vi "Dresden R2R Sputter 03.02.2018 IY24.vi"() -> ()   [LabVIEW 2009] (continued)
                                tunnel: [FALSE TRUE] -> w23599
                                frame #0 {
                                n20852 = local write "Ch3_Ch_vbv_do"(TRUE ("Ch1_Ch_cc_on_off_di")) -> ()
                                n20853 = Wait Until Next ms Multiple(millisecond multiple=u32 500) -> ()  [unwired: 1 out]
                                }
                                frame #1 {
                                }
                                }
                                n20854 = local read "Semi"() -> (w23600:bool)
                                n20855 = Or(x=w23599, y=w23600) -> (x .or. y?=w23598:bool)
                                }
                                }
                                frame #1 {
                                }
                                }
                                }
                                frame #1 {
                                n20856 = local read "Semi"() -> (w23610:bool)
                                n20857 = case shown="False" w23610 {
                                frame #0 {
                                n20858 = local write "Ch3_Sd13"(TRUE ("Ch1_Sd12")) -> ()
                                n20859 = Wait (ms)(milliseconds to wait=u32 1000) -> ()  [unwired: 1 out]
                                }
                                frame #1 {
                                }
                                }
                                }
                                }
                                }
                                frame #1 {
                                }
                                }
                                }
                                }
                              }
                              frame #13 {
                                # "TRNS GV-BP2 OPEN"
                                n20860 = local read "Yes 3"() -> (w23613:bool)
                                n20861 = case shown="True" w23613 {
                                frame #0 {
                                }
                                frame #1 {
                                n20862 = local read "Semi"() -> (w23614:bool)
                                n20863 = case shown="False" w23614 {
                                frame #0 {
                                n20864 = stacked-sequence {
                                frame #0 {
                                n20865 = local read "Semi"() -> (w23615:bool)
                                n20866 = case shown="False" w23615 {
                                frame #0 {
                                n20867 = while {
                                i -> [w23623]
                                stop <- w23620 stop-if-true
                                n20868 = Greater?(x=w23623, y=800) -> (0:w23622:bool)
                                n20869 = case shown="True" w23622 {
                                frame #0 {
                                }
                                frame #1 {
                                n20870 = local write "Error Message"("Shut Down process was cancelled.\nPlease check Trns GV-BP2\n connections." ("Error Message")) -> ()
                                n20871 = local write "Semi"(TRUE ("Semi")) -> ()
                                }
                                }
                                n20872 = local read "Ch3_pressure"() -> (w23618:dbl)
                                n20873 = Greater Or Equal?(x=w23618, y=700.0) -> (x >= y?=w23616:bool)
                                n20874 = case shown="True" w23616 {
                                tunnel: [FALSE w23627] -> w23619
                                frame #0 {
                                n20875 = Wait Until Next ms Multiple(millisecond multiple=u32 500) -> ()  [unwired: 1 out]
                                }
                                frame #1 {
                                n20876 = local read "Ch3_Trns_gv_bp2_di"() -> (w23628:bool)
                                n20877 = case shown="False" w23628 {
                                tunnel: [FALSE TRUE] -> w23627
                                frame #0 {
                                n20878 = local write "Ch3_Trns_gv_bp2_do"(TRUE ("Ch1_Trns_gv_bp2_do")) -> ()
                                n20879 = Wait Until Next ms Multiple(millisecond multiple=u32 500) -> ()  [unwired: 1 out]
                                }
                                frame #1 {
                                }
                                }
                                }
                                }
                                n20880 = local read "Semi"() -> (w23621:bool)
                                n20881 = Or(x=w23619, y=w23621) -> (x .or. y?=w23620:bool)
                                }
                                }
                                frame #1 {
                                }
                                }
                                }
                                frame #1 {
                                n20882 = local read "Semi"() -> (w23635:bool)
                                n20883 = case shown="False" w23635 {
                                frame #0 {
                                n20884 = local write "Ch3_Sd14"(TRUE ("Ch2_Sd0 14")) -> ()
                                n20885 = Wait (ms)(milliseconds to wait=u32 1000) -> ()  [unwired: 1 out]
                                }
                                frame #1 {
                                }
                                }
                                }
                                frame #2 {
                                n20886 = local read "Semi"() -> (w23638:bool)
                                n20887 = case shown="False" w23638 {
                                frame #0 {
                                n20888 = Wait (ms)(milliseconds to wait=u32 2000) -> ()  [unwired: 1 out]
                                }
                                frame #1 {
                                }
                                }
                                }
                                }
                                }
                                frame #1 {
                                }
                                }
                                }
                                }
                              }
                              frame #14 {
                                # "TRNS GV-BP OPEN"
                                n20889 = local read "Yes 3"() -> (w23640:bool)
                                n20890 = case shown="True" w23640 {
                                frame #0 {
                                }
                                frame #1 {
                                n20891 = local read "Semi"() -> (w23641:bool)
                                n20892 = case shown="False" w23641 {
                                frame #0 {
                                n20893 = stacked-sequence {
                                frame #0 {
                                n20894 = local read "Semi"() -> (w23642:bool)
                                n20895 = case shown="False" w23642 {
                                frame #0 {
                                n20896 = while {
                                i -> [w23650]
                                stop <- w23647 stop-if-true
                                n20897 = Greater?(x=w23650, y=800) -> (0:w23649:bool)
                                n20898 = case shown="True" w23649 {
                                frame #0 {
                                }
                                frame #1 {
                                n20899 = local write "Error Message"("Shut Down process was cancelled.\nPlease check Trns GV-BP\n connections." ("Error Message")) -> ()
                                n20900 = local write "Semi"(TRUE ("Semi")) -> ()
                                }
                                }
                                n20901 = local read "Ch3_pressure"() -> (w23645:dbl)
                                n20902 = Greater Or Equal?(x=w23645, y=700.0) -> (x >= y?=w23643:bool)
                                n20903 = case shown="True" w23643 {
                                tunnel: [FALSE w23654] -> w23646
                                frame #0 {
                                n20904 = Wait Until Next ms Multiple(millisecond multiple=u32 500) -> ()  [unwired: 1 out]
                                }
                                frame #1 {
                                n20905 = local read "Ch3_Trns_gv_bp_di"() -> (w23655:bool)
                                n20906 = case shown="False" w23655 {
                                tunnel: [FALSE TRUE] -> w23654
                                frame #0 {
                                n20907 = local write "Ch3_Trns_gv_bp_do"(TRUE ("Ch1_Trns_gv_bp2_do")) -> ()
                                n20908 = Wait Until Next ms Multiple(millisecond multiple=u32 500) -> ()  [unwired: 1 out]
                                }
                                frame #1 {
                                }
                                }
                                }
                                }
                                n20909 = local read "Semi"() -> (w23648:bool)
                                n20910 = Or(x=w23646, y=w23648) -> (x .or. y?=w23647:bool)
                                }
                                }
                                frame #1 {
                                }
                                }
                                }
                                frame #1 {
                                n20911 = local read "Semi"() -> (w23662:bool)
                                n20912 = case shown="False" w23662 {
                                frame #0 {
                                n20913 = local write "Ch3_Sd15"(TRUE ("Ch2_Sd0 15")) -> ()
                                n20914 = Wait (ms)(milliseconds to wait=u32 1000) -> ()  [unwired: 1 out]
                                }
                                frame #1 {
                                }
                                }
                                }
                                frame #2 {
                                n20915 = local read "Semi"() -> (w23665:bool)
                                n20916 = case shown="False" w23665 {
                                frame #0 {
                                n20917 = Wait (ms)(milliseconds to wait=u32 2000) -> ()  [unwired: 1 out]
                                }
                                frame #1 {
                                }
                                }
                                }
                                }
                                }
                                frame #1 {
                                }
                                }
                                }
                                }
                              }
                              frame #15 {
                                # "CH-ATM OPEN &  CHECK"
                                n20918 = local read "Yes 3"() -> (w23667:bool)
                                n20919 = case shown="True" w23667 {
                                frame #0 {
                                }
                                frame #1 {
                                n20920 = local read "Semi"() -> (w23668:bool)
                                n20921 = case shown="False" w23668 {
                                frame #0 {
                                n20922 = stacked-sequence {
                                frame #0 {
                                n20923 = local read "Semi"() -> (w23669:bool)
                                n20924 = case shown="False" w23669 {
                                frame #0 {
                                n20925 = while {
                                i -> [w23675]
                                stop <- w23672 stop-if-true
                                n20926 = Greater?(x=w23675, y=1700) -> (0:w23674:bool)
                                n20927 = case shown="True" w23674 {
                                frame #0 {
                                }
                                frame #1 {
                                n20928 = local write "Error Message"("Shut Down process was cancelled.\nPlease check Chamber \nvacuum connections." ("Error Message")) -> ()
                                n20929 = local write "Semi"(TRUE ("Semi")) -> ()
                                }
                                }
                                n20930 = local read "Ch3_Ch_atm_di"() -> (w23671:bool)
                                n20931 = case shown="False" w23671 {
                                tunnel: [FALSE TRUE] -> w23670
                                frame #0 {
                                n20932 = Wait Until Next ms Multiple(millisecond multiple=u32 500) -> ()  [unwired: 1 out]
                                }
                                frame #1 {
                                }
                                }
                                n20933 = local read "Semi"() -> (w23673:bool)
                                n20934 = Or(x=w23670, y=w23673) -> (x .or. y?=w23672:bool)
                                }
                                }
                                frame #1 {
                                }
                                }
                                }
                                frame #1 {
                                n20935 = local read "Semi"() -> (w23682:bool)
                                n20936 = case shown="False" w23682 {
                                frame #0 {
                                n20937 = local write "Ch3_Sd16"(TRUE ("Ch1_Sd10")) -> ()
                                n20938 = Wait (ms)(milliseconds to wait=u32 1000) -> ()  [unwired: 1 out]
                                }
                                frame #1 {
                                }
                                }
                                }
                                frame #2 {
                                n20939 = local read "Semi"() -> (w23685:bool)
                                n20940 = case shown="False" w23685 {
                                frame #0 {
                                n20941 = Wait (ms)(milliseconds to wait=u32 2000) -> ()  [unwired: 1 out]
                                }
                                frame #1 {
                                }
                                }
                                }
                                }
                                }
                                frame #1 {
                                }
                                }
                                }
                                }
                              }
                              frame #16 {
                                # "TRNS GV-BP2 close"
                                n20942 = local read "Semi"() -> (w23687:bool)
                                n20943 = case shown="False" w23687 {
                                frame #0 {
                                n20944 = stacked-sequence {
                                frame #0 {
                                n20945 = local read "Semi"() -> (w23688:bool)
                                n20946 = case shown="False" w23688 {
                                frame #0 {
                                n20947 = while {
                                i -> [w23694]
                                stop <- w23690 stop-if-true
                                n20948 = Greater?(x=w23694, y=50) -> (0:w23693:bool)
                                n20949 = case shown="True" w23693 {
                                frame #0 {
                                }
                                frame #1 {
                                n20950 = local write "Error Message"("Shut Down Process  cancelled\nbecause  Trns-GV-BP2  not closed.\nPlease check Trns GV-BP2 connections." ("Error Message")) -> ()
                                n20951 = local write "Semi"(TRUE ("Semi")) -> ()
                                }
                                }
                                n20952 = local read "Ch3_Trns_gv_bp2_di"() -> (w23689:bool)
                                n20953 = case shown="True" w23689 {
                                tunnel: [TRUE FALSE] -> w23691
                                frame #0 {
                                }
                                frame #1 {
                                n20954 = Wait Until Next ms Multiple(millisecond multiple=u32 500) -> ()  [unwired: 1 out]
                                n20955 = local write "Ch3_Trns_gv_bp2_do"(FALSE ("Ch1_Ch_cc_on_off_di")) -> ()
                                }
                                }
                                n20956 = local read "Semi"() -> (w23692:bool)
                                n20957 = Or(x=w23691, y=w23692) -> (x .or. y?=w23690:bool)
                                }
                                }
                                frame #1 {
                                }
                                }
                                }
                                frame #1 {
                                n20958 = local read "Semi"() -> (w23702:bool)
                                n20959 = case shown="False" w23702 {
                                frame #0 {
                                n20960 = local write "Ch3_Sd17"(TRUE ("Ch1_Sd10 3")) -> ()
                                n20961 = Wait (ms)(milliseconds to wait=u32 1000) -> ()  [unwired: 1 out]
                                }
                                frame #1 {
                                }
                                }
                                }
                                }
                                }
                                frame #1 {
                                }
                                }
                              }
                              frame #17 {
                                # "TRNS GV-BP close"
                                n20962 = local read "Semi"() -> (w23705:bool)
                                n20963 = case shown="False" w23705 {
                                frame #0 {
                                n20964 = stacked-sequence {
                                frame #0 {
                                n20965 = local read "Semi"() -> (w23706:bool)
                                n20966 = case shown="False" w23706 {
                                frame #0 {
                                n20967 = while {
                                i -> [w23712]
                                stop <- w23708 stop-if-true
                                n20968 = Greater?(x=w23712, y=50) -> (0:w23711:bool)
                                n20969 = case shown="True" w23711 {
                                frame #0 {
                                }
                                frame #1 {
                                n20970 = local write "Error Message"("Shut Down Process  cancelled\nbecause  Trns-GV-BP  not closed.\nPlease check Trns-GV-BP connections." ("Error Message")) -> ()
                                n20971 = local write "Semi"(TRUE ("Semi")) -> ()
                                }
                                }
                                n20972 = local read "Ch3_Trns_gv_bp_di"() -> (w23707:bool)
                                n20973 = case shown="True" w23707 {
                                tunnel: [TRUE FALSE] -> w23709
                                frame #0 {
                                }
                                frame #1 {
                                n20974 = Wait Until Next ms Multiple(millisecond multiple=u32 500) -> ()  [unwired: 1 out]
                                n20975 = local write "Ch3_Trns_gv_bp_do"(FALSE ("Ch1_Ch_cc_on_off_di")) -> ()
                                }
                                }
                                n20976 = local read "Semi"() -> (w23710:bool)
                                n20977 = Or(x=w23709, y=w23710) -> (x .or. y?=w23708:bool)
                                }
                                }
                                frame #1 {
                                }
                                }
                                }
                                frame #1 {
                                n20978 = local read "Semi"() -> (w23720:bool)
                                n20979 = case shown="False" w23720 {
                                frame #0 {
                                n20980 = local write "Ch3_Sd18"(TRUE ("Ch1_Sd10 3")) -> ()
                                n20981 = Wait (ms)(milliseconds to wait=u32 1000) -> ()  [unwired: 1 out]
                                }
                                frame #1 {
                                }
                                }
                                }
                                }
                                }
                                frame #1 {
                                }
                                }
                              }
                              frame #18 {
                                # "CH-VBV CLOSE &  CHECK"
                                n20982 = local read "Yes 3"() -> (w23723:bool)
                                n20983 = case shown="True" w23723 {
                                frame #0 {
                                }
                                frame #1 {
                                n20984 = local read "Semi"() -> (w23724:bool)
                                n20985 = case shown="False" w23724 {
                                frame #0 {
                                n20986 = stacked-sequence {
                                frame #0 {
                                n20987 = local read "Semi"() -> (w23725:bool)
                                n20988 = case shown="False" w23725 {
                                frame #0 {
                                n20989 = while {
                                i -> [w23735]
                                stop <- w23731 stop-if-true
                                n20990 = Greater?(x=w23735, y=50) -> (0:w23734:bool)
                                n20991 = case shown="True" w23734 {
                                frame #0 {
                                }
                                frame #1 {
                                n20992 = local write "Error Message"("Shut Down Process  cancelled\nbecause  CH-VBV  not closed.\nPlease check CH-VB3 connections." ("Error Message")) -> ()
                                n20993 = local write "Semi"(TRUE ("Semi")) -> ()
                                }
                                }
                                n20994 = local read "Tp3_speed_gui"() -> (w23729:i32)
                                n20995 = local read "Yes 3"() -> (w23728:bool)
                                n20996 = Greater Or Equal?(x=w23729, y=u64 100) -> (x >= y?=w23727:bool)
                                n20997 = And(x=w23728, y=w23727) -> (x .and. y?=w23726:bool)
                                n20998 = case shown="True" w23726 {
                                tunnel: [TRUE w23738] -> w23732
                                frame #0 {
                                }
                                frame #1 {
                                n20999 = local read "Ch3_Ch_vbv_di"() -> (w23739:bool)
                                n21000 = case shown="True" w23739 {
                                tunnel: [TRUE FALSE] -> w23738
                                frame #0 {
                                }
                                frame #1 {
                                n21001 = Wait Until Next ms Multiple(millisecond multiple=u32 500) -> ()  [unwired: 1 out]
                                n21002 = local write "Ch3_Ch_vbv_do"(FALSE ("Ch1_Ch_cc_on_off_di")) -> ()
                                }
                                }
                                }
                                }
                                n21003 = local read "Semi"() -> (w23733:bool)
                                n21004 = Or(x=w23732, y=w23733) -> (x .or. y?=w23731:bool)
                                }
                                }
                                frame #1 {
                                }
                                }
                                }
                                frame #1 {
                                n21005 = local read "Semi"() -> (w23746:bool)
                                n21006 = case shown="False" w23746 {
                                frame #0 {
                                n21007 = local write "Ch3_Sd19"(TRUE ("Ch1_Sd10 2")) -> ()
                                n21008 = Wait (ms)(milliseconds to wait=u32 1000) -> ()  [unwired: 1 out]
                                }
                                frame #1 {
                                }
                                }
                                }
                                frame #2 {
                                n21009 = local read "Semi"() -> (w23749:bool)
                                n21010 = case shown="False" w23749 {
                                frame #0 {
                                n21011 = Wait (ms)(milliseconds to wait=u32 3000) -> ()  [unwired: 1 out]
                                }
                                frame #1 {
                                }
                                }
                                }
                                }
                                }
                                frame #1 {
                                }
                                }
                                }
                                }
                              }
                              frame #19 {
                                # "CLOSE PC-BV"
                                n21012 = local read "Yes 3"() -> (w23751:bool)
                                n21013 = case shown="True" w23751 {
                                frame #0 {
                                }
                                frame #1 {
                                n21014 = local read "Semi"() -> (w23752:bool)
                                n21015 = case shown="False" w23752 {
                                frame #0 {
                                n21016 = stacked-sequence {
                                frame #0 {
                                n21017 = local read "Semi"() -> (w23753:bool)
                                n21018 = case shown="False" w23753 {
                                frame #0 {
                                n21019 = stacked-sequence {
                                frame #0 {
                                n21020 = local read "Semi"() -> (w23754:bool)
                                n21021 = case shown="False" w23754 {
                                frame #0 {
                                n21022 = local write "Pc_bv3_auto_close"(TRUE ("Tp1_auto_start")) -> ()
                                }
                                frame #1 {
                                }
                                }
                                }
                                frame #1 {
                                n21023 = local read "Semi"() -> (w23756:bool)
                                n21024 = case shown="False" w23756 {
                                frame #0 {
                                n21025 = Wait (ms)(milliseconds to wait=u32 1000) -> ()  [unwired: 1 out]
                                }
                                frame #1 {
                                }
                                }
                                }
                                frame #2 {
                                n21026 = local read "Semi"() -> (w23758:bool)
                                n21027 = case shown="False" w23758 {
                                frame #0 {
                                n21028 = while {
                                i -> [w23764]
                                stop <- w23760 stop-if-true
                                n21029 = local read "Pc_bv_closed_ch3"() -> (w23762:bool)
                                n21030 = Greater?(x=w23764, y=120) -> (0:w23763:bool)
                                n21031 = local read "Semi"() -> (w23761:bool)
                                n21032 = Compound Arithmetic op=OR(w23761, w23762, w23763) -> (w23760:bool)
                                n21033 = Wait (ms)(milliseconds to wait=u32 500) -> ()  [unwired: 1 out]
                                }
                                }
                                frame #1 {
                                }
                                }
                                }
                                frame #3 {
                                n21034 = local read "Semi"() -> (w23766:bool)
                                n21035 = case shown="False" w23766 {
                                frame #0 {
                                n21036 = local read "Pc_bv_closed_ch3"() -> (w23767:bool)
                                n21037 = case shown="False" w23767 {
                                frame #0 {
                                n21038 = local write "Pc_bv3_auto_close"(TRUE ("Pc_bv1_auto_open")) -> ()
                                }
                                frame #1 {
                                }
                                }
                                }
                                frame #1 {
                                }
                                }
                                }
                                frame #4 {
                                n21039 = local read "Semi"() -> (w23769:bool)
                                n21040 = case shown="False" w23769 {
                                frame #0 {
                                n21041 = local read "Pc_bv_closed_ch3"() -> (w23770:bool)
                                n21042 = case shown="False" w23770 {
                                frame #0 {
                                n21043 = Wait (ms)(milliseconds to wait=u32 1000) -> ()  [unwired: 1 out]
                                }
                                frame #1 {
                                }
                                }
                                }
                                frame #1 {
                                }
                                }
                                }
                                frame #5 {
                                n21044 = local read "Semi"() -> (w23772:bool)
                                n21045 = case shown="False" w23772 {
                                frame #0 {
                                n21046 = while {
                                i -> [w23778]
                                stop <- w23774 stop-if-true
                                n21047 = local read "Pc_bv_closed_ch3"() -> (w23776:bool)
                                n21048 = Greater?(x=w23778, y=120) -> (0:w23777:bool)
                                n21049 = local read "Semi"() -> (w23775:bool)
                                n21050 = Compound Arithmetic op=OR(w23775, w23776, w23777) -> (w23774:bool)
                                n21051 = Wait (ms)(milliseconds to wait=u32 500) -> ()  [unwired: 1 out]
                                }
                                }
                                frame #1 {
                                }
                                }
                                }
                                frame #6 {
                                n21052 = local read "Semi"() -> (w23780:bool)
                                n21053 = case shown="False" w23780 {
                                frame #0 {
                                n21054 = local read "Pc_bv_closed_ch3"() -> (w23781:bool)
                                n21055 = case shown="False" w23781 {
                                frame #0 {
                                n21056 = local write "Error Message"("Shut Down process  cancelled\nbecause  PC-BV not closed.\nPlease check PC-BV3 connections." ("Error Message")) -> ()
                                n21057 = Wait (ms)(milliseconds to wait=u32 1000) -> ()  [unwired: 1 out]
                                }
                                frame #1 {
                                }
                                }
                                }
                                frame #1 {
                                }
                                }
                                }
                                }
                                }
                                frame #1 {
                                }
                                }
                                }
                                frame #1 {
                                n21058 = local read "Semi"() -> (w23784:bool)
                                n21059 = case shown="False" w23784 {
                                frame #0 {
                                n21060 = Wait (ms)(milliseconds to wait=u32 1000) -> ()  [unwired: 1 out]
                                n21061 = local write "Ch3_Sd20"(TRUE ("Ch1_Sd14")) -> ()
                                }
                                frame #1 {
                                }
                                }
                                }
                                }
                                }
                                frame #1 {
                                }
                                }
                                }
                                }
                              }
                              frame #20 {
                                # "CH-VBV CLOSE &  CHECK"
                                n21062 = local read "Semi"() -> (w23787:bool)
                                n21063 = case shown="False" w23787 {
                                frame #0 {
                                n21064 = stacked-sequence {
                                frame #0 {
                                n21065 = local read "Semi"() -> (w23788:bool)
                                n21066 = case shown="False" w23788 {
                                frame #0 {
                                n21067 = while {
                                i -> [w23794]
                                stop <- w23790 stop-if-true
                                n21068 = Greater?(x=w23794, y=50) -> (0:w23793:bool)
                                n21069 = case shown="True" w23793 {
                                frame #0 {
                                }
                                frame #1 {
                                n21070 = local write "Error Message"("Shut Down Process  cancelled\nbecause  CH-VBV  not closed.\nPlease check CH-VBV3 connections." ("Error Message")) -> ()
                                n21071 = local write "Semi"(TRUE ("Semi")) -> ()
                                }
                                }
                                n21072 = local read "Ch3_Ch_vbv_di"() -> (w23789:bool)
                                n21073 = case shown="True" w23789 {
                                tunnel: [TRUE FALSE] -> w23791
                                frame #0 {
                                }
                                frame #1 {
                                n21074 = Wait Until Next ms Multiple(millisecond multiple=u32 500) -> ()  [unwired: 1 out]
                                n21075 = local write "Ch3_Ch_vbv_do"(FALSE ("Ch1_Ch_cc_on_off_di")) -> ()
                                }
                                }
                                n21076 = local read "Semi"() -> (w23792:bool)
                                n21077 = Or(x=w23791, y=w23792) -> (x .or. y?=w23790:bool)
                                }
                                }
                                frame #1 {
                                }
                                }
                                }
                                frame #1 {
                                n21078 = local read "Semi"() -> (w23802:bool)
                                n21079 = case shown="False" w23802 {
                                frame #0 {
                                n21080 = local write "Ch3_Sd21"(TRUE ("Ch1_Sd10 3")) -> ()
                                n21081 = Wait (ms)(milliseconds to wait=u32 1000) -> ()  [unwired: 1 out]
                                }
                                frame #1 {
                                }
                                }
                                }
                                }
                                }
                                frame #1 {
                                }
                                }
                              }
                              frame #21 {
                                # "FINISH SHUTDOWN"
                                n21082 = local read "Semi"() -> (w23805:bool)
                                n21083 = case shown="False" w23805 {
                                frame #0 {
                                n21084 = stacked-sequence {
                                frame #0 {
                                n21085 = local read "Semi"() -> (w23806:bool)
                                n21086 = case shown="False" w23806 {
                                frame #0 {
                                w23807 = TRUE ("Visible")
                                n21087 = property on="final_mes_tab" class="TabCtl (strict)"("Visible"=w23807) -> ()  [unwired: 2 in, 2 out]
                                n21088 = local write "Cnt_Do_Buzzer"(w23807) -> ()
                                n21089 = local write "system_status"(" CH3 Shut Down Process was completed." ("system_status")) -> ()
                                n21090 = Wait (ms)(milliseconds to wait=u32 3000) -> ()  [unwired: 1 out]
                                }
                                frame #1 {
                                }
                                }
                                }
                                frame #1 {
                                n21091 = local read "Semi"() -> (w23810:bool)
                                n21092 = case shown="False" w23810 {
                                frame #0 {
                                w23811 = FALSE ("Visible")
                                n21093 = local write "Shutdown_ch3"(w23811) -> ()
                                n21094 = local write "Cnt_Do_Buzzer"(w23811) -> ()
                                n21095 = property on="final_mes_tab" class="TabCtl (strict)"("Visible"=w23811) -> ()  [unwired: 2 in, 2 out]
                                n21096 = local write "system_status"("" ("system_status")) -> ()
                                n21097 = Wait (ms)(milliseconds to wait=u32 3000) -> ()  [unwired: 1 out]
                                }
                                frame #1 {
                                }
                                }
                                }
                                frame #2 {
                                n21098 = local read "Semi"() -> (w23814:bool)
                                n21099 = case shown="False" w23814 {
                                frame #0 {
                                n21100 = stacked-sequence {
                                frame #0 {
                                n21101 = local write "Pps_code_entry"("PF233=" ("Pps_code_entry")) -> ()
                                }
                                frame #1 {
                                n21102 = Wait (ms)(milliseconds to wait=u32 500) -> ()  [unwired: 1 out]
                                }
                                frame #2 {
                                n21103 = local write "Ppsok"(TRUE ("Ppsok")) -> ()
                                }
                                frame #3 {
                                n21104 = Wait (ms)(milliseconds to wait=u32 500) -> ()  [unwired: 1 out]
                                }
                                }
                                }
                                frame #1 {
                                }
                                }
                                }
                                frame #3 {
                                n21105 = local read "Semi"() -> (w23819:bool)
                                n21106 = case shown="False" w23819 {
                                frame #0 {
                                n21107 = stacked-sequence {
                                frame #0 {
                                n21108 = local write "Pps_code_entry"("PF234=" ("Pps_code_entry")) -> ()
                                }
                                frame #1 {
                                n21109 = Wait (ms)(milliseconds to wait=u32 500) -> ()  [unwired: 1 out]
                                }
                                frame #2 {
                                n21110 = local write "Ppsok"(TRUE ("Ppsok")) -> ()
                                }
                                frame #3 {
                                n21111 = Wait (ms)(milliseconds to wait=u32 500) -> ()  [unwired: 1 out]
                                }
                                }
                                }
                                frame #1 {
                                }
                                }
                                }
                                frame #4 {
                                n21112 = local read "Semi"() -> (w23824:bool)
                                n21113 = case shown="False" w23824 {
                                frame #0 {
                                n21114 = local write "Ch3_Sd22"(TRUE ("Ch1_Sd15")) -> ()
                                n21115 = Wait (ms)(milliseconds to wait=u32 500) -> ()  [unwired: 1 out]
                                }
                                frame #1 {
                                }
                                }
                                }
                                }
                                }
                                frame #1 {
                                }
                                }
                              }
                            }
                          }
                        }
                      }
                    }
                  }
                  frame #1 {
                  }
                }
              }
            }
          }
          frame #1 {
          }
        }
      }
    }
    n21116 = case shown="True" "Start_up_ch4" {
      frame #0 {
      }
      frame #1 {
        # "START UP OF CH4 PROCEDURE"
        n21117 = stacked-sequence {
          frame #0 {
            # "ROUTINE CHECK"
            n21118 = local read "Semi"() -> (w22208:bool)
            n21119 = case shown="False" w22208 {
              frame #0 {
                n21120 = stacked-sequence {
                  frame #0 {
                    n21121 = local write "Clean_Pumping_ch4"(TRUE) -> ()
                    n21122 = local write "final_process_messages"("Start up process was completed." ("final_process_messages")) -> ()
                    n21123 = property on="Pressure_time_graph_ch4" class="WFChart (strict)"("History Data"=dbl[] []) -> ()  [unwired: 2 in, 2 out]
                    n21124 = local write "system_status"("Start up process continues." ("system_status")) -> ()
                    n21125 = Wait (ms)(milliseconds to wait=u32 1000) -> ()  [unwired: 1 out]
                  }
                  frame #1 {
                    n21126 = local read "Semi"() -> (w22214:bool)
                    n21127 = case shown="False" w22214 {
                      frame #0 {
                        n21128 = stacked-sequence {
                          frame #0 {
                            n21129 = local read "Semi"() -> (w22215:bool)
                            n21130 = case shown="False" w22215 {
                              frame #0 {
                                n21131 = while {
                                i -> [w22222]
                                stop <- w22218 stop-if-true
                                n21132 = Greater?(x=w22222, y=50) -> (0:w22216:bool)
                                n21133 = case shown="True" w22216 {
                                frame #0 {
                                }
                                frame #1 {
                                n21134 = local write "Error Message"("Start up process cancelled because\nthere is no enough air pressure.\nPlease check air pressure connections." ("Error Message")) -> ()